vi "UHR-Fleezers Control (host) - 10.4.vi"() -> ()   [LabVIEW 2010] (continued)
            n251 = Absolute Value(x=w2893) -> (abs(x)=w2881:dbl)
            n252 = Compound Arithmetic op=MULTIPLY(w2899, w2898, w2887) -> (w2894:u64)
            n253 = local write "wait to reset values"(w2909) -> ()
            n254 = local write "MCL Scanning"(w2909) -> ()
            n255 = Divide(x=w2894, y=w2881) -> (x/y=w2891:dbl)
            "MCL Count" <- w2891
            n256 = xnode "Read/Write Control"("FPGA VI Reference In"=w2908, "error in"=w2907, "Scan steps (MCL)"=w2881, "Number of scans (MCL)"=w2903, "Cycles per step (MCL)"=u64 1, "Scan freq.  increment (MCL)"=w2884, "1D or 2D Scan?"=w2904, "MCL Scan Axis"=w2904, "Cont. Scan (MCL)"=w2904, "MCL count"=w2891) -> ("FPGA VI Reference Out"=w2906:T20, "error out"=w2905:errorcluster)
            n257 = xnode "Read/Write Control"("FPGA VI Reference In"=w2906, "error in"=w2905, "AI to FIFO"=w2909, "APD to FIFO"=w2909, "Start scan"=w2909, "Start scan (MCL)"=w2909) -> ("FPGA VI Reference Out"=w2911:T20, "error out"=w2910:errorcluster)
          }
        }
        "Raster Scanning..." <- TRUE ("Scanning...")
      }
    }
    n258 = Subtract(x=w848, y=w853) -> (x-y=→"x-y 2":u32)
    n259 = And(x="Save scans", y=w1057) -> (x .and. y?=w1103:bool)
    n260 = Compound Arithmetic op=OR("Start MCL Scan", "Confocal Image", "Confocal Linescan") -> (w1055:bool)
    n261 = And(x="Save Data (MCL)", y=w1055) -> (x .and. y?=w1102:bool)
    n262 = case "Start MCL raster scan" shown="False" w1055 {
      tunnel: w1105 -> [w2126 w2141]
      tunnel: w1104 -> [w2125 w2140]
      tunnel: [w2126 w2136] -> w861
      tunnel: [w2125 w2135] -> w860
      tunnel: [FALSE w2134] -> w1088
      tunnel: "Start MCL Scan" -> [_ w2129]
      tunnel: "Confocal Image" -> [_ w2128]
      tunnel: "Confocal Linescan" -> [_ _]
      frame False {
      }
      frame True {
        w2134 = TRUE
        n263 = case shown="True" "Restart DMA? (MCL)" {
          tunnel: [w2386 w2388] -> w2139
          tunnel: [w2385 w2387] -> w2138
          tunnel: w2141 -> [w2386 w2391]
          tunnel: w2140 -> [w2385 w2390]
          frame False {
          }
          frame True {
            n264 = call "reset FPGA DMA.vi"("error in"=w2390, "FPGA VI Reference In"=w2391) -> ("error out"=w2387:errorcluster, "FPGA VI Reference Out"=w2388:T20)
            n265 = local write "Overflow (data lost)"(FALSE ("Overflow (data lost)")) -> ()
          }
        }
        n266 = case shown="False" w2129 {
          selector: w2129 -> [_ w2145]
          tunnel: w2128 -> [w2144 _]
          tunnel: [w2144 w2145] -> w2127
          frame False {
            n267 = property on="2D or 1D Scan" class="Bool (strict)"("Val(Sgnl)"=w2144) -> ()  [unwired: 2 in, 2 out]
            n268 = property on="Confocal Image" class="Bool (strict)"("Value"=FALSE ("Start Confocal Map")) -> ()  [unwired: 2 in, 2 out]
          }
          frame True {
          }
        }
        n269 = local write "MCL Scanning"(w2134) -> ()
        n270 = local read "AO1"() -> (w2131:dbl)
        n271 = local read "AO2"() -> (w2130:dbl)
        n272 = case shown="False" "Center Scan" {
          tunnel: w2139 -> [w2152 w2264]
          tunnel: w2138 -> [w2151 w2263]
          tunnel: [w2150 w2262] -> w2136
          tunnel: [w2149 w2261] -> w2135
          tunnel: [w2147 w2248] -> w2133
          tunnel: [w2146 w2247] -> w2132
          tunnel: w2131 -> [w2147 w2253]
          tunnel: w2130 -> [w2146 w2256]
          tunnel: w2127 -> [_ _]
          frame False {
            w2148 = TRUE ("AI to FIFO")
            n273 = xnode "Read/Write Control"("FPGA VI Reference In"=w2152, "error in"=w2151, "AI to FIFO"=w2148, "APD to FIFO"=w2148, "Start scan (MCL)"=w2148) -> ("FPGA VI Reference Out"=w2150:T20, "error out"=w2149:errorcluster)
          }
          frame True {
            w2260 = TRUE ("AI to FIFO")
            n274 = local read "Scan steps (MCL)"() -> (w2239:u64)
            n275 = local read "Scan lines (y)"() -> (w2235:u64)
            n276 = local read "Fast Scan Dir"() -> (w2246:bool)
            n277 = local read "Actual MCL Inc (V)"() -> (w2236:dbl)
            n278 = Decrement(x=w2235) -> (x-1=w2234:u64)
            n279 = Decrement(x=w2239) -> (x-1=w2238:u64)
            n280 = Multiply(x=w2236, y=w2234) -> (x*y=w2233:dbl)
            n281 = Divide(x=w2233, y=2.0) -> (x/y=w2243:dbl)
            n282 = Multiply(x=w2236, y=w2238) -> (x*y=w2237:dbl)
            n283 = Divide(x=w2237, y=2.0) -> (x/y=w2242:dbl)
            n284 = Select(t=w2242, s=w2246, f=w2243) -> (s? t:f=w2241:dbl)
            n285 = Select(t=w2243, s=w2246, f=w2242) -> (s? t:f=w2245:dbl)
            n286 = Subtract(x=w2253, y=w2245) -> (x-y=w2244:dbl)
            n287 = Subtract(x=w2256, y=w2241) -> (x-y=w2240:dbl)
            n288 = local read "2D or 1D Scan"() -> (w2258:bool)
            n289 = Not(x=w2246) -> (.not. x?=w2252:bool)
            n290 = Not(x=w2258) -> (.not. x?=w2254:bool)
            n291 = And(x=w2246, y=w2254) -> (x .and. y?=w2255:bool)
            n292 = And(x=w2254, y=w2252) -> (x .and. y?=w2257:bool)
            n293 = Select(t=w2256, s=w2257, f=w2240) -> (s? t:f=w2247:dbl)
            n294 = Select(t=w2253, s=w2255, f=w2244) -> (s? t:f=w2248:dbl)
            n295 = call "Volt to I16.vi"("Voltage In"=w2248) -> ("I16 Voltage Out"=w2251:i16)
            n296 = call "Volt to I16.vi"("Voltage In"=w2247) -> ("I16 Voltage Out"=w2250:i16)
            n297 = xnode "Read/Write Control"("FPGA VI Reference In"=w2264, "error in"=w2263, "AI to FIFO"=w2260, "APD to FIFO"=w2260, "Start scan (MCL)"=w2260, "AO1"=w2251, "AO2"=w2250) -> ("FPGA VI Reference Out"=w2262:T20, "error out"=w2261:errorcluster)
          }
        }
        "Initial Y" <- w2133
        "Initial X" <- w2132
        "wait to reset values" <- w2134
      }
    }
    n298 = local read "Trap Pos Elements/DMA read"() -> (w936:u32)
    n299 = local read "Trap AI Elements/DMA read"() -> (w859:u32)
    n300 = local read "APD Elements/DMA read"() -> (w979:u32)
    n301 = local read "Trap AI FIFO Depth"() -> (w1152:u32)
    n302 = xnode "Get APD Data"("FPGA VI Reference In"=w861, "error in"=w860, "Number of Elements"=w979, "Timeout (ms)"=-1) -> ("Data"=w978:u32[], "Elements Remaining"=→"APD FIFO Elements Remaining":u32)  [unwired: 2 out]
    n303 = xnode "Invoke Method"("FPGA VI Reference In"=w861, "error in"=w860, "Number of Elements"=w936, "Timeout (ms)"=-1) -> ("Data"=w900:u16[], "Elements Remaining"=→"Trap Pos FIFO El Remaining":u32)  [unwired: 2 out]
    n304 = xnode "Invoke Method"("FPGA VI Reference In"=w861, "error in"=w860, "Number of Elements"=w859, "Timeout (ms)"=-1 ("Timeout")) -> ("FPGA VI Reference Out"=w863:T20, "error out"=w862:errorcluster, "Data"=w865:i16[], "Elements Remaining"=w864:u32)
    "Trap AI FIFO El. Rem." <- w864
    n305 = Subtract(x=w1152, y=u32 0) -> (x-y=w1151:u32)
    n306 = Decimate 1D Array(w900) -> (w897:u16[], w899:u16[], w898:u16[])
    n307 = Divide(x=w864, y=w1151) -> (x/y=w1150:dbl)
    "Buffer Status" <- w1150
    n308 = To Unsigned Long Integer(number=w897) -> (unsigned 32bit integer=w896:u32[])
    n309 = Join Numbers(hi=w899, lo=w898) -> ((hi.lo)=w895:u32[])
    n310 = Equal?(x=w1150, y=1.0) -> (x = y?=w1148:bool)
    n311 = Join Numbers(hi=w896, lo=w895) -> ((hi.lo)=w889:u64[])
    n312 = call "IR AOM word to freq - vec.vi"("Frequency Word In (double vec)"=w889) -> ("Frequency Out"=w935:dbl[])
    n313 = case "Alert buffer overflow" shown="True" w1148 {
      frame False {
      }
      frame True {
        n314 = call <vilib>:"Beep.vi"() -> ()  [unwired: 3 in, 9 out]
        "Overflow (data lost)" <- TRUE ("Overflow (data lost)")
      }
    }
    n315 = Decimate 1D Array(w935) -> (w934:dbl[], w933:dbl[])
    n316 = Build Array(w934, w933) -> (w932:dbl[][])
    n317 = local read "Trap Sets"() -> (w1016:u32)
    n318 = case "Deinterlace trap data, average down PSD" shown="1, Default" w1016 {
      tunnel: w865 -> [w2421 w2486]
      tunnel: [w2418 w2483] -> w1009
      tunnel: [w2421 w2485] -> w892
      tunnel: "Detector Type" -> [w2420 w2481]
      tunnel: [w2419 w2484] -> w1008
      tunnel: [w2417 w2482] -> w1123
      frame 1, Default {
        n319 = Divide(x=w2421, y=3276.7) -> (x/y=w2422:dbl[])
        n320 = Decimate 1D Array(w2422) -> (w2431:dbl[], w2430:dbl[], w2429:dbl[], w2428:dbl[], w2427:dbl[], w2426:dbl[], w2425:dbl[], w2424:dbl[])
        n321 = case shown="\"IR-QPD + PSD + FB-QPD position\"" w2420 {
          tunnel: w2431 -> [w2455 w2480]
          tunnel: w2430 -> [w2454 w2479]
          tunnel: w2429 -> [w2439 w2457]
          tunnel: w2428 -> [w2440 w2467]
          tunnel: w2427 -> [w2453 w2478]
          tunnel: w2426 -> [w2452 w2477]
          tunnel: w2425 -> [w2436 w2458]
          tunnel: w2424 -> [w2435 w2456]
          tunnel: [w2434 w2464] -> w2419
          tunnel: [w2433 w2463] -> w2418
          tunnel: [w2432 w2462] -> w2417
          frame "IR-QPD + PSD + FB-QPD", Default {
            w2432 = 0  # Channel pattern
            n322 = Divide(x=w2455, y=w2440) -> (x/y=w2442:dbl[])
            n323 = Divide(x=w2454, y=w2440) -> (x/y=w2441:dbl[])
            n324 = Divide(x=w2453, y=w2436) -> (x/y=w2438:dbl[])
            n325 = Divide(x=w2452, y=w2435) -> (x/y=w2437:dbl[])
            n326 = Build Array(w2442, w2441, w2440, w2439, w2438, w2437, w2436, w2435) -> (w2433:dbl[][])
            n327 = Bundle("T1 Y", "T1 X", "T1 Sum", "FB Sum", "PSD Y", "PSD X", "PSD Y Sum", "PSD X Sum") -> (w2451:T39)  [unwired: 1 out]
            n328 = Cluster To Array(cluster=w2451) -> (array=w2434:string[])
          }
          frame "IR-QPD + PSD + FB-QPD position" {
            w2462 = 3  # Channel pattern
            n329 = Negate(x=w2458) -> (-x=w2459:dbl[])
            n330 = Divide(x=w2480, y=w2467) -> (x/y=w2469:dbl[])
            n331 = Divide(x=w2479, y=w2467) -> (x/y=w2468:dbl[])
            n332 = Divide(x=w2478, y=w2458) -> (x/y=w2466:dbl[])
            n333 = Divide(x=w2477, y=w2459) -> (x/y=w2465:dbl[])
            n334 = Build Array(w2469, w2468, w2467, w2456, w2457, w2466, w2465, w2458) -> (w2463:dbl[][])
            n335 = Bundle("T1 Y", "T1 X", "T1 Sum", "FB X", "FB Sum", "PSD Y", "PSD X", "PSD Y Sum") -> (w2476:T39)  [unwired: 1 out]
            n336 = Cluster To Array(cluster=w2476) -> (array=w2464:string[])
          }
        }
      }
      frame 2 {
        n337 = case shown="\"IR-QPD + PSD + FB-QPD X position\"" w2481 {
          tunnel: w2486 -> [w2548 w2615 w2686]
          tunnel: [w2487 w2606 w2617] -> w2485
          tunnel: [w2514 w2597 w2664] -> w2484
          tunnel: [w2513 w2560 w2631] -> w2483
          tunnel: [w2507 w2595 w2662] -> w2482
          frame "IR-QPD + PSD + FB-QPD", Default {
            w2507 = 1  # Channel pattern
            # "time average x2 the 4th signal and the 4 psd signals (detection laser)"
            # "deinterlace 3 signals from qpd"
            n338 = Decimate 1D Array(w2548) -> (w2547:i16[], w2546:i16[], w2512:i16[], w2545:i16[], w2535:i16[], w2533:i16[], w2532:i16[], w2530:i16[])
            n339 = Decimate 1D Array(w2512) -> (w2511:i16[], w2510:i16[])
            n340 = Decimate 1D Array(w2547) -> (w2544:i16[], w2516:i16[])
            n341 = Decimate 1D Array(w2546) -> (w2543:i16[], w2541:i16[])
            n342 = Decimate 1D Array(w2545) -> (w2542:i16[], w2540:i16[])
            n343 = call "downsample 1D array - double.vi"("Ave N"=2.0, "Array In"=w2535) -> ("Array Out"=w2534:dbl[])  [unwired: 1 out]
            n344 = call "downsample 1D array - double.vi"("Ave N"=2.0, "Array In"=w2533) -> ("Array Out"=w2515:dbl[])  [unwired: 1 out]
            n345 = call "downsample 1D array - double.vi"("Ave N"=2.0, "Array In"=w2532) -> ("Array Out"=w2531:dbl[])  [unwired: 1 out]
            n346 = call "downsample 1D array - double.vi"("Ave N"=2.0, "Array In"=w2530) -> ("Array Out"=w2529:dbl[])  [unwired: 1 out]
            n347 = Interleave 1D Arrays(w2544, w2543, w2542, w2516, w2541, w2540, w2511, w2510, w2534, w2515, w2531, w2529) -> (w2528:dbl[])
            n348 = Divide(x=w2528, y=3276.7) -> (x/y=w2527:dbl[])
            n349 = Decimate 1D Array(w2527) -> (w2526:dbl[], w2525:dbl[], w2524:dbl[], w2523:dbl[], w2522:dbl[], w2521:dbl[], w2509:dbl[], w2508:dbl[], w2520:dbl[], w2519:dbl[], w2518:dbl[], w2517:dbl[])
            n350 = Divide(x=w2526, y=w2524) -> (x/y=w2494:dbl[])
            n351 = Divide(x=w2525, y=w2524) -> (x/y=w2493:dbl[])
            n352 = Divide(x=w2523, y=w2521) -> (x/y=w2492:dbl[])
            n353 = Divide(x=w2522, y=w2521) -> (x/y=w2491:dbl[])
            n354 = Divide(x=w2520, y=w2518) -> (x/y=w2490:dbl[])
            n355 = Divide(x=w2519, y=w2517) -> (x/y=w2489:dbl[])
            n356 = Build Array(w2494, w2493, w2524, w2492, w2491, w2521, w2509, w2508, w2490, w2489, w2518, w2517) -> (w2513:dbl[][])
            n357 = Bundle("T1 Y", "T1 X", "T1 Sum", "T2 Y", "T2 X", "T2 Sum", "T1 FB Sum", "T2 FB Sum", "PSD Y", "PSD X", "PSD Y Sum", "PSD X Sum") -> (w2495:T40)  [unwired: 1 out]
            n358 = To Word Integer(number=w2528) -> (16bit integer=w2487:i16[])
            n359 = Cluster To Array(cluster=w2495) -> (array=w2514:string[])
          }
          frame "IR-QPD + PSD + FB-QPD X position" {
            w2595 = 2  # Channel pattern
            # "time average x2 the 3 psd signals (detection laser)"
            # "deinterlace 3 signals from qpds"
            n360 = Decimate 1D Array(w2615) -> (w2614:i16[], w2613:i16[], w2596:i16[], w2612:i16[], w2558:i16[], w2555:i16[], w2552:i16[], w2583:i16[])
            n361 = Decimate 1D Array(w2596) -> (w2581:i16[], w2579:i16[])
            n362 = Decimate 1D Array(w2614) -> (w2611:i16[], w2598:i16[])
            n363 = Decimate 1D Array(w2613) -> (w2610:i16[], w2608:i16[])
            n364 = Decimate 1D Array(w2612) -> (w2609:i16[], w2607:i16[])
            n365 = Decimate 1D Array(w2583) -> (w2582:i16[], w2580:i16[])
            n366 = call "downsample 1D array - I16.vi"("Ave N"=2.0, "Array In"=w2558) -> ("Array Out"=w2556:i16[])  [unwired: 1 in]
            n367 = call "downsample 1D array - I16.vi"("Ave N"=2.0, "Array In"=w2552) -> ("Array Out"=w2550:i16[])  [unwired: 1 in]
            n368 = call "downsample 1D array - I16.vi"("Ave N"=2.0, "Array In"=w2555) -> ("Array Out"=w2553:i16[])  [unwired: 1 in]
            n369 = Interleave 1D Arrays(w2611, w2610, w2609, w2598, w2608, w2607, w2582, w2581, w2580, w2579, w2556, w2553, w2550) -> (w2606:i16[])
            n370 = Divide(x=w2606, y=3276.7) -> (x/y=w2605:dbl[])
            n371 = Decimate 1D Array(w2605) -> (w2604:dbl[], w2603:dbl[], w2602:dbl[], w2601:dbl[], w2600:dbl[], w2599:dbl[], w2571:dbl[], w2569:dbl[], w2568:dbl[], w2566:dbl[], w2565:dbl[], w2564:dbl[], w2561:dbl[])
            n372 = Negate(x=w2561) -> (-x=w2559:dbl[])
            n373 = Divide(x=w2565, y=w2561) -> (x/y=w2563:dbl[])
            n374 = Divide(x=w2564, y=w2559) -> (x/y=w2562:dbl[])
            n375 = Divide(x=w2604, y=w2602) -> (x/y=w2587:dbl[])
            n376 = Divide(x=w2603, y=w2602) -> (x/y=w2586:dbl[])
            n377 = Divide(x=w2601, y=w2599) -> (x/y=w2585:dbl[])
            n378 = Divide(x=w2600, y=w2599) -> (x/y=w2584:dbl[])
            n379 = Divide(x=w2571, y=w2569) -> (x/y=w2570:dbl[])
            n380 = Divide(x=w2568, y=w2566) -> (x/y=w2567:dbl[])
            n381 = Build Array(w2587, w2586, w2602, w2585, w2584, w2599, w2570, w2569, w2567, w2566, w2563, w2562, w2561) -> (w2560:dbl[][])
            n382 = Bundle("T1 Y", "T1 X", "T1 Sum", "T2 Y", "T2 X", "T2 Sum", "T1 FB X", "T1 FB Sum", "T2 FB X", "T2 FB Sum", "PSD Y", "PSD X", "PSD Y Sum") -> (w2588:T41)  [unwired: 1 out]
            n383 = Cluster To Array(cluster=w2588) -> (array=w2597:string[])
          }
          frame "IR-QPD + PSD + FB-QPD XY positions" {
            w2662 = 4  # Channel pattern
            # "time average x2 the 3 psd signals (detection laser)"
            # "deinterlace 3 signals from qpds"
            n384 = Decimate 1D Array(w2686) -> (w2685:i16[], w2684:i16[], w2663:i16[], w2683:i16[], w2629:i16[], w2675:i16[], w2674:i16[], w2651:i16[])
            n385 = Decimate 1D Array "Feedback Sum"(w2663) -> (w2647:i16[], w2645:i16[])
            n386 = Decimate 1D Array "QPD Y"(w2685) -> (w2682:i16[], w2665:i16[])
            n387 = Decimate 1D Array "QPD X"(w2684) -> (w2681:i16[], w2679:i16[])
            n388 = Decimate 1D Array "Feedback Y"(w2629) -> (w2628:i16[], w2627:i16[])
            n389 = Decimate 1D Array "QPD Sum"(w2683) -> (w2680:i16[], w2678:i16[])
            n390 = Decimate 1D Array "Feedback X"(w2651) -> (w2648:i16[], w2646:i16[])
            n391 = call "downsample 1D array - double.vi"("Ave N"=2.0, "Array In"=w2675) -> ("Array Out"=w2650:dbl[])  [unwired: 1 out]
            n392 = call "downsample 1D array - double.vi"("Ave N"=2.0, "Array In"=w2674) -> ("Array Out"=w2649:dbl[])  [unwired: 1 out]
            n393 = Interleave 1D Arrays(w2682, w2681, w2680, w2665, w2679, w2678, w2628, w2648, w2647, w2627, w2646, w2645, w2650, w2649) -> (w2673:dbl[])
            n394 = Divide(x=w2673, y=3276.7) -> (x/y=w2672:dbl[])
            n395 = Decimate 1D Array(w2672) -> (w2671:dbl[], w2670:dbl[], w2669:dbl[], w2668:dbl[], w2667:dbl[], w2666:dbl[], w2624:dbl[], w2638:dbl[], w2622:dbl[], w2623:dbl[], w2636:dbl[], w2620:dbl[], w2634:dbl[], w2632:dbl[])
            n396 = Negate(x=w2632) -> (-x=w2630:dbl[])
            n397 = Divide(x=w2634, y=w2630) -> (x/y=w2633:dbl[])
            n398 = Divide(x=w2623, y=w2620) -> (x/y=w2619:dbl[])
            n399 = Divide(x=w2624, y=w2622) -> (x/y=w2621:dbl[])
            n400 = Divide(x=w2671, y=w2669) -> (x/y=w2655:dbl[])
            n401 = Divide(x=w2670, y=w2669) -> (x/y=w2654:dbl[])
            n402 = Divide(x=w2668, y=w2666) -> (x/y=w2653:dbl[])
            n403 = Divide(x=w2667, y=w2666) -> (x/y=w2652:dbl[])
            n404 = Divide(x=w2638, y=w2622) -> (x/y=w2637:dbl[])
            n405 = Divide(x=w2636, y=w2620) -> (x/y=w2635:dbl[])
            n406 = Build Array(w2655, w2654, w2669, w2653, w2652, w2666, w2621, w2637, w2622, w2619, w2635, w2620, w2633, w2632) -> (w2631:dbl[][])
            n407 = Bundle("T1 Y", "T1 X", "T1 Sum", "T2 Y", "T2 X", "T2 Sum", "T1 FB Y", "T1 FB X", "T1 FB Sum", "T2 FB Y", "T2 FB X", "T2 FB Sum", "PSD X", "PSD Y Sum") -> (w2618:T42)  [unwired: 1 out]
            n408 = To Word Integer(number=w2673) -> (16bit integer=w2617:i16[])
            n409 = Cluster To Array(cluster=w2618) -> (array=w2664:string[])
          }
        }
      }
    }
    "AI labels" <- w1008
    n410 = Decimate 1D Array(w978) -> (w1006:u32[], w942:u32[])
    n411 = local read "DMA Update Period (s)"() -> (w1017:dbl)
    n412 = local read "BD 1 Frequency 2 (MHz)"() -> (w884:dbl)
    n413 = local read "BD 1 Frequency 1 (MHz)"() -> (w885:dbl)
    n414 = Build Array(w1006, w942) -> (w1085:u32[][])
    n415 = local read "Data Period (s)"() -> (w991:dbl)
    n416 = Decimate 1D Array(w892) -> (w915:i16[], w914:i16[], w912:i16[], w911:i16[])  [unwired: 9 out]
    n417 = To Double Precision Float(number=w1085) -> (double precision float=w1086:dbl[][])
    n418 = local read "APD Integration Time (s)"() -> (w955:dbl)
    n419 = Divide(x=w915, y=w914) -> (x/y=w916:dbl[])
    n420 = Divide(x=w912, y=w911) -> (x/y=w913:dbl[])
    n421 = feedback #1(0.0) -> (w929:dbl)
    n422 = Add(x=w1017, y=w929) -> (x+y=w1125:dbl)
    n423 = feedback-in #1(w1125) -> ()
    n424 = local read "AOM X Cal (nm/MHz)"() -> (w882:dbl)
    n425 = To Time Stamp(1:w929) -> (0:w928:timestamp)
    n426 = Split 1D Array(array=w916, index="N El. to Ave.") -> (second subarray=w919:dbl[])  [unwired: 1 out]
    n427 = Split 1D Array(array=w913, index="N El. to Ave.") -> (second subarray=w918:dbl[])  [unwired: 1 out]
    n428 = local read "Trap X AI1 (DMA)"() -> (w917:T14)
    n429 = Multiply(x=w991, y="Trap Disp. Downsample") -> (x*y=w930:dbl)
    "Display Period (s)" <- w930
    n430 = Bundle("BD 1 Frequency 1 (MHz)"=w885, "BD 1 Frequency 2 (MHz)"=w884) -> (w886:T43)  [unwired: 1 out]
    n431 = for "Trap AI" {
      tunnel: [w2416] -> w1119 mode=indexing
      tunnel: w928 -> [w2406]
      tunnel: "Trap Disp. Downsample" -> [w2414]
      tunnel: w1009 -> [w2412] mode=indexing
      tunnel: w991 -> [w2411]
      tunnel: w1008 -> [w2410] mode=indexing
      tunnel: w927 -> [w2409]
      tunnel: [w2408] -> w966 mode=indexing
      tunnel: w930 -> [w2407]
      workers-P: _ -> [_]
      n432 = Bundle By Name("Y"=w2412, "dt"=w2411) -> (w2413:waveform(dbl))  [unwired: 1 out]
      n433 = Set Waveform Attribute(5:w2410, 6:w2409, 7:w2413) -> (3:w2408:waveform(dbl))  [unwired: 1 in, 2 out]
      n434 = call "downsample 1D array - double.vi"("Ave N"=w2414, "Array In"=w2412) -> ("Array Out"=w2415:dbl[])  [unwired: 1 out]
      n435 = Bundle By Name(cluster=w2408, "t0"=w2406, "Y"=w2415, "dt"=w2407) -> (w2416:waveform(dbl))
    }
    n436 = call <vilib>:"Mean.vi"("X"=w918) -> ("mean"=w906:dbl)  [unwired: 1 out]
    n437 = call <vilib>:"Mean.vi"("X"=w919) -> ("mean"=w907:dbl)  [unwired: 1 out]
    n438 = Cluster To Array(cluster=w886) -> (array=w883:dbl[])
    n439 = Reciprocal(x=w930) -> (1/x=→"Trap Disp. Freq. (Hz)":dbl)
    n440 = local read "Data points/scans (MCL)"() -> (w1097:dbl)
    n441 = To Fixed-Point(number=w906) -> (fixed-point=w904:fxp<+/-,16,1>)  [unwired: 1 in]
    n442 = To Fixed-Point(number=w907) -> (fixed-point=w905:fxp<+/-,16,1>)  [unwired: 1 in]
    n443 = Bundle("Trap 1 Pos.", "Trap 2 Pos.") -> (w926:cluster{string, string})  [unwired: 1 out]
    n444 = Bundle By Name(cluster=w917, "Set 1"=w905, "Set 2"=w904) -> (→"Trap X AI1 (DMA)":T14)
    n445 = Cluster To Array(cluster=w926) -> (array=w923:string[])
    n446 = for "Trap Position" {
      tunnel: w932 -> [w1321] mode=indexing
      tunnel: "Trap Disp. Downsample" -> [w1320]
      tunnel: w930 -> [w1318]
      tunnel: w928 -> [w1317]
      tunnel: w927 -> [w1315]
      tunnel: w923 -> [w1314] mode=indexing
      tunnel: [w1313] -> w881 mode=indexing
      tunnel: w883 -> [w1311] mode=indexing
      tunnel: w882 -> [w1309]
      n447 = call "downsample 1D array - double.vi"("Ave N"=w1320, "Array In"=w1321) -> ("Array Out"=w1319:dbl[])  [unwired: 1 out]
      n448 = Subtract(x=w1319, y=w1311) -> (x-y=w1312:dbl[])
      n449 = Multiply(x=w1309, y=w1312) -> (x*y=w1310:dbl[])
      n450 = Bundle By Name("Y"=w1310, "dt"=w1318, "t0"=w1317) -> (w1316:waveform(dbl))  [unwired: 1 out]
      n451 = Set Waveform Attribute(5:w1314, 6:w1315, 7:w1316) -> (3:w1313:waveform(dbl))  [unwired: 1 in, 2 out]
    }
    "Trap Positions" <- w881
    n452 = Bundle("APD 1", "APD 2") -> (w1118:cluster{string, string})  [unwired: 1 out]
    n453 = Cluster To Array(cluster=w1118) -> (array=w1115:string[])
    n454 = for "APD" {
      tunnel: w1086 -> [w2395] mode=indexing
      tunnel: w955 -> [w2403]
      tunnel: [w2399] -> w962 mode=indexing
      tunnel: "APD Disp. Scale" -> [w2400]
      tunnel: w927 -> [w2398]
      tunnel: w1115 -> [w2397] mode=indexing
      tunnel: "APD Disp. Downsample" -> [w2393]
      tunnel: [w2396] -> w1114
      workers-P: _ -> [_]
      tunnel: w928 -> [w2392]
      n455 = call "integrate 1D array interval - double.vi"("Ave N"=w2393, "Array In"=w2395) -> ("Array Out"=w2394:dbl[])  [unwired: 1 out]
      n456 = Multiply(x=w2403, y=w2393) -> (x*y=w2396:dbl)
      n457 = Divide(x=w2394, y=w2400) -> (x/y=w2401:dbl[])
      n458 = Bundle By Name("t0"=w2392, "Y"=w2401, "dt"=w2396) -> (w2402:waveform(dbl))  [unwired: 1 out]
      n459 = Set Waveform Attribute(5:w2397, 6:w2398, 7:w2402) -> (3:w2399:waveform(dbl))  [unwired: 1 in, 2 out]
    }
    "APD Display Period (s)" <- w1114
    n460 = Reciprocal(x=w1114) -> (1/x=→"APD Display Freq. (Hz)":dbl)
    n461 = local read "Display Period (s)"() -> (w990:dbl)
    n462 = Increment(x=w1097) -> (x+1=w1098:dbl)
    n463 = Index Array(array=w881, index=0) -> (element=w879:waveform(dbl))
    n464 = To Double Precision Float(number=w1006) -> (double precision float=w1005:dbl[])
    n465 = feedback #2(w1098) -> (w1101:dbl)
    n466 = Select(t=0, s=w1088, f=w1101) -> (s? t:f=w1094:dbl)
    n467 = Array Size(array=w1005) -> (size(s)=w1100:i32)
    n468 = Add(x=w1100, y=w1094) -> (x+y=w1095:dbl)
    n469 = Unbundle By Name(w879) -> ("Y"=w877:dbl[])
    n470 = feedback #3(w1006) -> (w1084:u32[])
    n471 = Build Array (concatenate)(w1084, w1006) -> (w1081:u32[])
    n472 = feedback #4(w942) -> (w961:u32[])
    n473 = Divide(x="Bead Sep. Int. Time (s)", y=w990) -> (x/y=w875:dbl)
    n474 = Build Array (concatenate)(w961, w942) -> (w960:u32[])
    n475 = Greater?(x=w1095, y=w1097) -> (0:w1096:bool)
    n476 = feedback #5(w877) -> (w878:dbl[])
    n477 = Build Array (concatenate)(w877, w878) -> (w876:dbl[])
    n478 = Select(t=w1094, s=w1096, f=w1095) -> (s? t:f=w1093:dbl)
    n479 = feedback-in #2(w1093) -> ()
    n480 = Array Size(array=w1081) -> (size(s)=w1078:i32)
    n481 = Array Size(array=w1006) -> (size(s)=w1080:i32)
    n482 = local read "MCL Scanning"() -> (w1091:bool)
    n483 = local read "APD Integration Time (s)"() -> (w969:dbl)
    n484 = Build Array (concatenate)(w962, w1119) -> (w964:waveform(dbl)[])
    "All Signals" <- w964
    n485 = Split 1D Array(array=w876, index=w875) -> (first subarray=w869:dbl[])  [unwired: 1 out]
    n486 = feedback-in #5(w869) -> ()
    n487 = Multiply(x=w1080, y="APD Ave N") -> (x*y=w1079:dbl)
    n488 = Greater?(x=w1078, y=w1079) -> (0:w1082:bool)
    n489 = Not(x=w1096) -> (.not. x?=w1090:bool)
    n490 = To Double Precision Float(number=w942) -> (double precision float=w941:dbl[])
    n491 = call <vilib>:"Mean.vi"("X"=w869) -> ("mean"=w868:dbl)  [unwired: 1 out]
    "Mean T1 Position (nm)" <- w868
    n492 = Subtract(x=w869, y=w868) -> (x-y=w874:dbl[])
    n493 = Square(x=w874) -> (x^2=w873:dbl[])
    n494 = And(x=w1090, y=w1091) -> (x .and. y?=w1092:bool)
    n495 = call <vilib>:"Mean.vi"("X"=w873) -> ("mean"=w872:dbl)  [unwired: 1 out]
    n496 = case shown="True" w1082 {
      tunnel: w1081 -> [w1976 w1983]
      tunnel: [w1976 w1981] -> w1022
      tunnel: w1079 -> [_ w1978]
      tunnel: w1078 -> [_ w1982]
      tunnel: w960 -> [w1975 w1980]
      tunnel: [w1975 w1977] -> w957
      frame False {
      }
      frame True {
        n497 = Subtract(x=w1982, y=w1978) -> (x-y=w1979:dbl)
        n498 = Array Subset(array=w1983, index=w1979, length=w1978) -> (w1981:u32[])
        n499 = Array Subset(array=w1980, index=w1979, length=w1978) -> (w1977:u32[])
      }
    }
    n500 = feedback-in #3(w1022) -> ()
    n501 = feedback-in #4(w957) -> ()
    n502 = Or(x=w1092, y=w1088) -> (x .or. y?=w1089:bool)
    n503 = Square Root(x=w872) -> (sqrt(x)=w871:dbl)
    n504 = Equal?(x="Tab Control 6", y=T30."High Res Display") -> (x = y?=w1012:bool)
    n505 = Multiply(x="APD Disp. Scale", y=w962) -> (x*y=w971:waveform(dbl)[])
    n506 = Multiply(x="APD Disp. Downsample", y=w969) -> (x*y=w967:dbl)
    n507 = Multiply(x=10.0, y=w871) -> (x*y=→"Trap 1 Position RMS (A)":dbl)
    n508 = Divide(x=w971, y=w967) -> (x/y=w939:waveform(dbl)[])
    n509 = Index Array(array=w939, index=0) -> (element=w949:waveform(dbl))
    n510 = case "For computing FFTs for display" shown="True" "Compute FFT" {
      tunnel: w966 -> [_ w3239]
      frame False {
      }
      frame True {
        n511 = Build Array("FFT 1 Choice 1", "FFT 1 Choice 2", "FFT 2 Choice 1", "FFT 2 Choice 2") -> (w3232:u16[])
        n512 = Array Size(array=w3239) -> (size(s)=w3238:i32)
        n513 = feedback-in #6(w3232) -> ()
        n514 = feedback #6(u16[] [100, 100, 100, 100]) -> (w3233:u16[])
        n515 = feedback-in #7("# Spectra to Ave.") -> ()
        n516 = feedback #7("# Spectra to Ave.") -> (w3230:dbl)
        n517 = Not Equal?(x="# Spectra to Ave.", y=w3230) -> (x != y?=w3229:bool)
        n518 = Not Equal?(x=w3232, y=w3233) -> (x != y?=w3231:bool)
        n519 = feedback #8(1.0) -> (w3216:dbl)
        n520 = Compound Arithmetic op=OR("Reset FFT", w3231, w3229) -> (w3214:bool)
        n521 = Select(t=1.0, s=w3214, f=w3216) -> (s? t:f=w3218:dbl)
        n522 = Greater?(x=w3218, y="# Spectra to Ave.") -> (0:w3237:bool)
        n523 = Increment(x=w3218) -> (x+1=w3217:dbl)
        n524 = feedback-in #8(w3217) -> ()
        n525 = local read "DMA Update Period (s)"() -> (w3212:dbl)
        n526 = Multiply(x="# Spectra to Ave.", y=w3212) -> (x*y=→"Ave. Time (s)":dbl)
        n527 = Build Array(cluster{"f0":dbl, "df":dbl, "magnitude":dbl[]} {"f0"=0.0, "df"=0.0, "magnitude"=[]} ("PSD")) -> (w3221:cluster{"f0":dbl, "df":dbl, "magnitude":dbl[]}[])
        n528 = Build Array(w3221, w3221, w3221, w3221) -> (w3223:T44)
        n529 = feedback #9(w3223) -> (w3228:T44)
        n530 = for {
          N: 4 -> [_]
          tunnel: w3232 -> [w3261] mode=indexing
          tunnel: w3239 -> [w3262]
          tunnel: w3238 -> [w3264]
          tunnel: w3214 -> [w3257]
          tunnel: w3237 -> [w3256]
          tunnel: "# Spectra to Ave." -> [w3255]
          tunnel: [w3254] -> w3227 mode=indexing
          tunnel: w3228 -> [w3259] mode=indexing
          tunnel: [w3258] -> w3215 mode=indexing
          tunnel: w3218 -> [w3253]
          n531 = Less?(x=w3261, y=w3264) -> (x < y?=w3263:bool)
          n532 = Index Array(array=w3262, index=w3261) -> (element=w3260:waveform(dbl))
          n533 = case shown="True" w3263 {
            tunnel: w3260 -> [_ w3281]
            tunnel: w3259 -> [w3266 w3279]
            tunnel: [w3266 w3267] -> w3258
            tunnel: w3257 -> [_ w3278]
            tunnel: w3256 -> [_ w3271]
            tunnel: w3255 -> [_ w3270]
            tunnel: [cluster{"f0":dbl, "df":dbl, "magnitude":dbl[]} {"f0"=0.0, "df"=0.0, "magnitude"=[]} ("PSD") w3272] -> w3254
            tunnel: w3253 -> [_ w3269]
            frame False {
            }
            frame True {
              n534 = call <vilib>:"Std Deviation and Variance.vi"("X"=w3281) -> ("mean"=w3282:dbl)  [unwired: 1 in, 2 out]
              n535 = Subtract(x=w3281, y=w3282) -> (x-y=w3280:waveform(dbl))
              n536 = xnode "Spectral Measurements"("Signals"=w3280) -> ("PSD"=w3274:cluster{"f0":dbl, "df":dbl, "magnitude":dbl[]})  [unwired: 1 in, 1 out]
              n537 = case shown="False" w3278 {
                tunnel: w3279 -> [w3291 _]
                tunnel: [w3287 w3296] -> w3267
                tunnel: w3274 -> [w3290 w3297]
                tunnel: w3271 -> [w3289 _]
                frame False {
                  n538 = Build Array (concatenate)(w3291, w3290) -> (w3288:cluster{"f0":dbl, "df":dbl, "magnitude":dbl[]}[])
                  n539 = case shown="True" w3289 {
                    tunnel: w3288 -> [w3292 w3295]
                    tunnel: [w3292 w3293] -> w3287
                    frame False {
                    }
                    frame True {
                      n540 = Delete From Array(array=w3295, index=0) -> (array with subset deleted=w3293:cluster{"f0":dbl, "df":dbl, "magnitude":dbl[]}[])  [unwired: 1 in, 1 out]
                    }
                  }
                }
                frame True {
                  n541 = Build Array(w3297) -> (w3296:cluster{"f0":dbl, "df":dbl, "magnitude":dbl[]}[])
                }
              }
              n542 = for {
                tunnel: w3267 -> [w3286] mode=indexing
                tunnel: [w3285] -> w3277 mode=indexing
                workers-P: _ -> [_]
                n543 = Unbundle By Name(w3286) -> ("magnitude"=w3285:dbl[])
              }
              n544 = Transpose 2D Array(2D array=w3277) -> (transposed array=w3276:dbl[][])
              n545 = for {
                tunnel: w3276 -> [w3284] mode=indexing
                tunnel: [w3283] -> w3275 mode=indexing
                workers-P: _ -> [_]
                n546 = Add Array Elements(numeric array=w3284) -> (sum=w3283:dbl)
              }
              n547 = Select(t=w3270, s=w3271, f=w3269) -> (s? t:f=w3268:dbl)
              n548 = Divide(x=w3275, y=w3268) -> (x/y=w3273:dbl[])
              n549 = Bundle By Name(cluster=w3274, "magnitude"=w3273) -> (w3272:cluster{"f0":dbl, "df":dbl, "magnitude":dbl[]})
            }
          }
        }
        n550 = case shown="True" w3214 {
          tunnel: w3215 -> [w3246 w3252]
          tunnel: [w3246 w3247] -> w3213
          frame False {
          }
          frame True {
            n551 = Array Subset(array=w3252, index (row)=0 ("index"), length (row)=4 ("length"), index (col)=0 ("index"), length (col)=1 ("length")) -> (w3247:T44)
          }
        }
        n552 = feedback-in #9(w3213) -> ()
        n553 = Split 1D Array(array=w3227, index=2) -> (first subarray=→"FFT 1":cluster{"f0":dbl, "df":dbl, "magnitude":dbl[]}[], second subarray=→"FFT 2":cluster{"f0":dbl, "df":dbl, "magnitude":dbl[]}[])
      }
    }
    n554 = Index Array(array=w939, index=1) -> (element=w947:waveform(dbl))
    n555 = case "For displaying the high resolution display (no downsampling)" shown="True" w1012 {
      tunnel: w966 -> [_ w1485]
      frame False {
      }
      frame True {
        n556 = Index Array(array=w1485, index="High Res. Display") -> (element=w1486:waveform(dbl))
        n557 = call <vilib>:"Std Deviation and Variance.vi"("X"=w1486) -> ("mean"=w1493:dbl, "standard deviation"=w1498:dbl)  [unwired: 1 in, 1 out]
        "Mean Intensity" <- w1493
        "Sigma" <- w1498
        n558 = Subtract(x=w1486, y=w1493) -> (x-y=w1492:waveform(dbl))
        n559 = Select(t=w1492, s="Subtract mean", f=w1486) -> (s? t:f=→"1 Channel":waveform(dbl))
        n560 = Divide(x=w1498, y=w1493) -> (x/y=→"Sigma/Mean":dbl)
        n561 = feedback #10(1) -> (w1487:i32)
        n562 = Greater Or Equal?(x=w1487, y="Slow mean N ave.") -> (x >= y?=w1500:bool)
        n563 = Increment(x=w1487) -> (x+1=w1502:i32)
        n564 = Select(t=1, s=w1500, f=w1502) -> (s? t:f=w1489:i32)
        n565 = feedback-in #10(w1489) -> ()
        n566 = feedback #11() -> (w1490:waveform(dbl))  [unwired: 1 out]
        n567 = case shown="Default" w1487 {
          tunnel: [w1505 w1508] -> w1491
          tunnel: w1490 -> [w1507 _]
          tunnel: w1486 -> [w1506 w1508]
          frame Default {
            n568 = call-poly <vilib>:"Append Waveforms.vi"("waveform B"=w1506, "waveform A"=w1507) -> ("waveform out"=w1505:waveform(dbl))  [unwired: 1 in, 8 out]
          }
          frame 1 {
          }
        }
        n569 = feedback-in #11(w1491) -> ()
        n570 = case shown="True" w1500 {
          tunnel: w1491 -> [_ w1504]
          frame False {
          }
          frame True {
            n571 = call <vilib>:"Mean.vi"("X"=w1504) -> ("mean"=→"Slow mean":dbl)  [unwired: 1 out]
          }
        }
      }
    }
    n572 = case "For plotting results of scanning MCL" shown="True" w1089 {
      tunnel: w1088 -> [_ w2016]
      tunnel: w1005 -> [_ w2112]
      tunnel: w1097 -> [_ _]
      tunnel: w966 -> [_ w2086]
      tunnel: w941 -> [_ w2017]
      tunnel: w940 -> [_ w1990]
      frame False {
      }
      frame True {
        w1997 = u32 0 items=["Horizontal", "Vertical", "Central", "1st Diagonal", "2nd Diagonal"] ("Type of Symmetry")
        w2025 = u32 0 items=["Horizontal", "Vertical", "Central", "1st Diagonal", "2nd Diagonal"] ("Type of Symmetry")
        w2028 = u32 0 items=["Horizontal", "Vertical", "Central", "1st Diagonal", "2nd Diagonal"] ("Type of Symmetry")
        w2057 = u32 0 items=["Horizontal", "Vertical", "Central", "1st Diagonal", "2nd Diagonal"] ("Type of Symmetry")
        n573 = Index Array(array=w2086, index=10) -> (element=w2092:waveform(dbl))
        n574 = Index Array(array=w2086, index=11) -> (element=w2089:waveform(dbl))
        n575 = local read "Cycles/step (MCL)"() -> (w2042:u64)
        n576 = Index Array(array=w2086, index="Channel") -> (element=w2088:waveform(dbl))
        n577 = Unbundle(w1990) -> ("New Image"=w1989:T2, "New Image"=w1988:T2, "New Image"=w1987:T2, "New Image"=w1986:T2)
        n578 = Unbundle By Name(w2092) -> ("Y"=w2044:dbl[])
        n579 = Unbundle By Name(w2089) -> ("Y"=w2046:dbl[])
        n580 = Unbundle By Name(w2088) -> ("Y"=w2051:dbl[])
        n581 = call "downsample 1D array - double.vi"("Ave N"=w2042, "Array In"=w2044) -> ("Array Out"=w2043:dbl[])  [unwired: 1 out]
        n582 = call "downsample 1D array - double.vi"("Ave N"=w2042, "Array In"=w2046) -> ("Array Out"=w2045:dbl[])  [unwired: 1 out]
        n583 = call "downsample 1D array - double.vi"("Ave N"=w2042, "Array In"=w2051) -> ("Array Out"=w2050:dbl[])  [unwired: 1 out]
        n584 = feedback #12(w2112) -> (w2113:dbl[])
        n585 = Build Array (concatenate)(w2113, w2112) -> (w2094:dbl[])
        n586 = feedback #13(w2017) -> (w2019:dbl[])
        n587 = Build Array (concatenate)(w2019, w2017) -> (w2018:dbl[])
        n588 = local read "Scan steps (MCL)"() -> (w1999:u64)
        n589 = Select(t=w2112, s=w2016, f=w2094) -> (s? t:f=w2098:dbl[])
        n590 = feedback-in #12(w2098) -> ()
        n591 = Select(t=w2017, s=w2016, f=w2018) -> (s? t:f=w2000:dbl[])
        n592 = feedback-in #13(w2000) -> ()
        n593 = local read "Scan lines (y)"() -> (w1985:u64)
        n594 = local read "N APD Samp/step"() -> (w2001:dbl)
        n595 = feedback #14(w2043) -> (w2100:dbl[])
        n596 = Build Array (concatenate)(w2100, w2043) -> (w2091:dbl[])
        n597 = feedback #15(w2050) -> (w2110:dbl[])
        n598 = Build Array (concatenate)(w2110, w2050) -> (w2109:dbl[])
        n599 = feedback #16(w2045) -> (w2102:dbl[])
        n600 = Build Array (concatenate)(w2102, w2045) -> (w2103:dbl[])
        n601 = Select(t=w2043, s=w2016, f=w2091) -> (s? t:f=w2047:dbl[])
        n602 = feedback-in #14(w2047) -> ()
        n603 = Select(t=w2050, s=w2016, f=w2109) -> (s? t:f=w2049:dbl[])
        n604 = feedback-in #15(w2049) -> ()
        n605 = Select(t=w2045, s=w2016, f=w2103) -> (s? t:f=w2048:dbl[])
        n606 = feedback-in #16(w2048) -> ()
        n607 = Multiply(x=w1999, y=u64 2) -> (x*y=w1984:u64)
        n608 = call "integrate 1D array interval - double.vi"("Ave N"=w2001, "Array In"=w2000) -> ("Array Out"=w2012:dbl[])  [unwired: 1 out]
        n609 = call "integrate 1D array interval - double.vi"("Ave N"=w2001, "Array In"=w2098) -> ("Array Out"=w2097:dbl[])  [unwired: 1 out]
        n610 = Array Size(array=w2012) -> (size(s)=w2013:i32)
        n611 = Array Size(array=w2097) -> (size(s)=w2099:i32)
        n612 = Multiply(x=w1985, y=w1984) -> (x*y=w2015:u64)
        n613 = Multiply(x=w1985, y=w1984) -> (x*y=w2107:u64)
        n614 = call <vilib>:"Mean.vi"("X"=w2047) -> ("mean"=w2031:dbl)  [unwired: 1 out]
        n615 = Subtract(x=w2015, y=w2013) -> (x-y=w2006:u64)
        n616 = call <vilib>:"Mean.vi"("X"=w2049) -> ("mean"=w2036:dbl)  [unwired: 1 out]
        n617 = call <vilib>:"Mean.vi"("X"=w2048) -> ("mean"=w2034:dbl)  [unwired: 1 out]
        n618 = call <vilib>:"Mean.vi"("X"=w2012) -> ("mean"=w2003:dbl)  [unwired: 1 out]
        n619 = Subtract(x=w2107, y=w2099) -> (x-y=w2041:u64)
        n620 = call <vilib>:"Mean.vi"("X"=w2097) -> ("mean"=w2038:dbl)  [unwired: 1 out]
        n621 = Initialize Array(1.0 ("element"), w2006) -> (w2002:dbl[])
        n622 = Initialize Array(1.0 ("element"), w2041) -> (w2032:dbl[])
        n623 = Multiply(x=w2002, y=w2003) -> (x*y=w2004:dbl[])
        n624 = Multiply(x=w2032, y=w2034) -> (x*y=w2035:dbl[])
        n625 = Multiply(x=w2032, y=w2036) -> (x*y=w2037:dbl[])
        n626 = Multiply(x=w2032, y=w2031) -> (x*y=w2033:dbl[])
        n627 = Multiply(x=w2032, y=w2038) -> (x*y=w2039:dbl[])
        n628 = Build Array (concatenate)(w2047, w2033) -> (w2101:dbl[])
        n629 = Build Array (concatenate)(w2049, w2037) -> (w2105:dbl[])
        n630 = Build Array (concatenate)(w2048, w2035) -> (w2104:dbl[])
        n631 = Build Array (concatenate)(w2012, w2004) -> (w2014:dbl[])
        n632 = Build Array (concatenate)(w2097, w2039) -> (w2106:dbl[])
        n633 = Reshape Array(w2101, w1985, w1984) -> (w2067:dbl[][])
        n634 = Reshape Array(w2014, w1985, w1984) -> (w2010:dbl[][])
        n635 = Reshape Array(w2105, w1985, w1984) -> (w2059:dbl[][])
        n636 = Reshape Array(w2104, w1985, w1984) -> (w2074:dbl[][])
        n637 = Reshape Array(w2106, w1985, w1984) -> (w2084:dbl[][])
        n638 = Array Subset(array=w2074, index (col)=0 ("index"), length (col)=w1999) -> (w2079:dbl[][])  [unwired: 2 in]
        n639 = Array Subset(array=w2074, index (col)=w1999) -> (w2077:dbl[][])  [unwired: 3 in]
        n640 = Array Subset(array=w2059, index (col)=0 ("index"), length (col)=w1999) -> (w2065:dbl[][])  [unwired: 2 in]
        n641 = Array Subset(array=w2059, index (col)=w1999) -> (w2063:dbl[][])  [unwired: 3 in]
        n642 = Array Subset(array=w2010, index (col)=0 ("index"), length (col)=w1999) -> (w2009:dbl[][])  [unwired: 2 in]
        n643 = Array Subset(array=w2010, index (col)=w1999) -> (w2007:dbl[][])  [unwired: 3 in]
        n644 = Array Subset(array=w2084, index (col)=0 ("index"), length (col)=w1999) -> (w2083:dbl[][])  [unwired: 2 in]
        n645 = Array Subset(array=w2084, index (col)=w1999) -> (w2081:dbl[][])  [unwired: 3 in]
        n646 = Array Subset(array=w2067, index (col)=0 ("index"), length (col)=w1999) -> (w2072:dbl[][])  [unwired: 2 in]
        n647 = Array Subset(array=w2067, index (col)=w1999) -> (w2070:dbl[][])  [unwired: 3 in]
        n648 = for {
          tunnel: w2079 -> [w2121] mode=indexing
          tunnel: [w2120] -> w2078 mode=indexing
          workers-P: _ -> [_]
          n649 = Reverse 1D Array(array=w2121) -> (reversed array=w2120:dbl[])
        }
        n650 = for {
          tunnel: w2065 -> [w2117] mode=indexing
          tunnel: [w2116] -> w2064 mode=indexing
          workers-P: _ -> [_]
          n651 = Reverse 1D Array(array=w2117) -> (reversed array=w2116:dbl[])
        }
        n652 = for {
          tunnel: w2009 -> [w2115] mode=indexing
          tunnel: [w2114] -> w2008 mode=indexing
          workers-P: _ -> [_]
          n653 = Reverse 1D Array(array=w2115) -> (reversed array=w2114:dbl[])
        }
        n654 = for {
          tunnel: w2083 -> [w2123] mode=indexing
          tunnel: [w2122] -> w2082 mode=indexing
          workers-P: _ -> [_]
          n655 = Reverse 1D Array(array=w2123) -> (reversed array=w2122:dbl[])
        }
        n656 = for {
          tunnel: w2072 -> [w2119] mode=indexing
          tunnel: [w2118] -> w2071 mode=indexing
          workers-P: _ -> [_]
          n657 = Reverse 1D Array(array=w2119) -> (reversed array=w2118:dbl[])
        }
        n658 = Index Array(array=w2084, index (row)=0) -> (element=→"Waveform Graph":dbl[])  [unwired: 1 in]
        n659 = Add(x=w2078, y=w2077) -> (x+y=w2076:dbl[][])
        n660 = Add(x=w2064, y=w2063) -> (x+y=w2062:dbl[][])
        n661 = Add(x=w2008, y=w2007) -> (x+y=w1992:dbl[][])
        n662 = Add(x=w2082, y=w2081) -> (x+y=w2056:dbl[][])
        n663 = Add(x=w2071, y=w2070) -> (x+y=w2069:dbl[][])
        n664 = Divide(x=w2062, y=2) -> (x/y=w2060:dbl[][])
        n665 = Divide(x=w2076, y=2) -> (x/y=w2021:dbl[][])
        n666 = Divide(x=w2069, y=2) -> (x/y=w2023:dbl[][])
        n667 = To Single Precision Float(number=w2056) -> (single precision float=w2055:sgl[][])
        n668 = Transpose 2D Array(2D array=w2060) -> (transposed array=→"Data map":dbl[][])
        n669 = To Single Precision Float(number=w1992) -> (single precision float=w1996:sgl[][])
        n670 = To Single Precision Float(number=w2021) -> (single precision float=w2027:sgl[][])
        n671 = To Single Precision Float(number=w2023) -> (single precision float=w2024:sgl[][])
        n672 = call "IMAQ ArrayToImage"("Image Pixels (Float)"=w2055, "Image"=w1989) -> ("Image Out"=w2058:T2)  [unwired: 8 in, 1 out]
        n673 = call "IMAQ ArrayToImage"("Image Pixels (Float)"=w1996, "Image"=w1988) -> ("Image Out"=w1998:T2)  [unwired: 8 in, 1 out]
        n674 = call "IMAQ ArrayToImage"("Image Pixels (Float)"=w2027, "Image"=w1987) -> ("Image Out"=w2029:T2)  [unwired: 8 in, 1 out]
        n675 = call "IMAQ ArrayToImage"("Image Pixels (Float)"=w2024, "Image"=w1986) -> ("Image Out"=w2026:T2)  [unwired: 8 in, 1 out]
        n676 = call "IMAQ Symmetry"("Type of Symmetry"=w2057, "Image Src"=w2058) -> ("Image Dst Out"=w2053:T2)  [unwired: 3 in, 1 out]
        n677 = call "IMAQ Symmetry"("Type of Symmetry"=w1997, "Image Src"=w1998) -> ("Image Dst Out"=w1994:T2)  [unwired: 3 in, 1 out]
        n678 = call "IMAQ Symmetry"("Type of Symmetry"=w2028, "Image Src"=w2029) -> ("Image Dst Out"=→"Detection Laser X":T2)  [unwired: 3 in, 1 out]
        n679 = call "IMAQ Symmetry"("Type of Symmetry"=w2025, "Image Src"=w2026) -> ("Image Dst Out"=→"Detection Laser Y":T2)  [unwired: 3 in, 1 out]
        n680 = call "IMAQ Set Simple Calibration"("Calibration Axis Info"=T31 {"Origin Pixel"={"X"=0.0, "Y"=0.0}, "Angle Relative to Horizontal (deg)"=0.0, "Axis Reference"=0}, "Grid Descriptor"=T32 {"X Step"=0.3, "Y Step"=0.3, "Unit"=enum."Undefined"}, "Image"=w2053) -> ("Calibrated Image"=→"APD 1":T2)  [unwired: 7 in, 1 out]
        n681 = call "IMAQ Set Simple Calibration"("Calibration Axis Info"=T31 {"Origin Pixel"={"X"=0.0, "Y"=0.0}, "Angle Relative to Horizontal (deg)"=0.0, "Axis Reference"=0}, "Grid Descriptor"=T32 {"X Step"=0.3, "Y Step"=0.3, "Unit"=enum."Undefined"}, "Image"=w1994) -> ("Calibrated Image"=→"APD 2":T2)  [unwired: 7 in, 1 out]
      }
    }
    n682 = Subtract(x=w947, y="APD 2 Offset") -> (x-y=w944:waveform(dbl))
    n683 = Subtract(x=w949, y="APD 1 Offset") -> (x-y=w945:waveform(dbl))
    n684 = Index Array(array=w964, index=3) -> (element=w1033:waveform(dbl))
    n685 = Index Array(array=w964, index=6) -> (element=w1030:waveform(dbl))
    n686 = Build Array(w945, w944) -> (→"APD Chart":waveform(dbl)[])
    n687 = Array Size(array=w1022) -> (size(s)=w1077:i32)
    n688 = call <vilib>:"Std Deviation and Variance.vi"("X"=w957) -> ("standard deviation"=w956:dbl)  [unwired: 1 in, 2 out]
    n689 = Add Array Elements(numeric array=w957) -> (sum=w959:u32)
    n690 = Add Array Elements(numeric array=w1022) -> (sum=w1087:u32)
    n691 = call <vilib>:"Std Deviation and Variance.vi"("X"=w1022) -> ("standard deviation"=w1021:dbl)  [unwired: 1 in, 2 out]
    n692 = Divide(x="T1 offset_x (mV)", y=1000.0) -> (x/y=w1034:dbl)
    n693 = Divide(x=w956, y=w955) -> (x/y=w952:dbl)
    "Rate sigma (Hz) 2" <- w952
    n694 = Multiply(x=w955, y=w1077) -> (x*y=w958:dbl)
    "Int. Time (s)" <- w958
    n695 = Divide(x=w959, y=w958) -> (x/y=w953:dbl)
    "APD 2 Rate (Hz)" <- w953
    n696 = Divide(x=w1087, y=w958) -> (x/y=w1019:dbl)
    "APD 1 Rate (Hz)" <- w1019
    n697 = Divide(x=w1021, y=w955) -> (x/y=w1020:dbl)
    "Rate sigma (Hz)" <- w1020
    n698 = Divide(x=w952, y=w953) -> (x/y=→"Sigma/Mean 2":dbl)
    n699 = Divide(x=w1020, y=w1019) -> (x/y=→"Sigma/Mean":dbl)
    n700 = Divide(x="T2 offset_x (mV)", y=1000.0) -> (x/y=w1032:dbl)
    n701 = case shown="0, Default" "Calibration" {
      tunnel: "T1 alpha_x (nm/V)" -> [_ w1952 w1973]
      tunnel: "T1 kappa_x (pN/nm)" -> [_ _ w1963]
      tunnel: "T2 alpha_x (nm/V)" -> [_ w1951 w1971]
      tunnel: "T2 kappa_x (pN/nm)" -> [_ _ w1964]
      tunnel: w1033 -> [w1934 w1949 w1969]
      tunnel: w1030 -> [w1933 w1947 w1967]
      tunnel: [w1934 w1946 w1966] -> w1063
      tunnel: [w1933 w1945 w1965] -> w1062
      tunnel: ["T1 X (V)" ("Label.Text") "T1 X (nm)" ("Label.Text") "T1 X (pN)" ("Label.Text")] -> w1051
      tunnel: ["T2 X (V)" ("Label.Text") "T2 X (nm)" ("Label.Text") "T2 X (pN)" ("Label.Text")] -> w1050
      tunnel: ["Position (V)" ("Label.Text") "Position (nm)" ("Label.Text") "Force (pN)" ("Label.Text")] -> w1052
      tunnel: w1032 -> [_ w1937 w1956]
      tunnel: w1034 -> [_ w1940 w1958]
      tunnel: ["Mean (V)" ("Label.Text") "Mean (nm)" ("Label.Text") "Mean (pN)" ("Label.Text")] -> w1047
      tunnel: ["Difference (V)" ("Label.Text") "Difference (nm)" ("Label.Text") "Difference (pN)" ("Label.Text")] -> w972
      frame 0, Default {
      }
      frame 1 {
        n702 = Unbundle By Name(w1949) -> ("Y"=w1953:dbl[])
        n703 = Unbundle By Name(w1947) -> ("Y"=w1938:dbl[])
        n704 = Subtract(x=w1953, y=w1940) -> (x-y=w1941:dbl[])
        n705 = Subtract(x=w1938, y=w1937) -> (x-y=w1939:dbl[])
        n706 = Multiply(x=w1939, y=w1951) -> (x*y=w1948:dbl[])
        n707 = Multiply(x=w1952, y=w1941) -> (x*y=w1950:dbl[])
        n708 = Bundle By Name(cluster=w1947, "Y"=w1948) -> (w1945:waveform(dbl))
        n709 = Bundle By Name(cluster=w1949, "Y"=w1950) -> (w1946:waveform(dbl))
      }
      frame 2 {
        n710 = Unbundle By Name(w1969) -> ("Y"=w1974:dbl[])
        n711 = Unbundle By Name(w1967) -> ("Y"=w1972:dbl[])
        n712 = Subtract(x=w1972, y=w1956) -> (x-y=w1957:dbl[])
        n713 = Subtract(x=w1974, y=w1958) -> (x-y=w1959:dbl[])
        n714 = Compound Arithmetic op=MULTIPLY(w1957, w1971, w1964) -> (w1968:dbl[])
        n715 = Compound Arithmetic op=MULTIPLY(w1963, w1973, w1959) -> (w1970:dbl[])
        n716 = Bundle By Name(cluster=w1967, "Y"=w1968) -> (w1965:waveform(dbl))
        n717 = Bundle By Name(cluster=w1969, "Y"=w1970) -> (w1966:waveform(dbl))
      }
    }
    n718 = feedback-in #17("Calibration") -> ()
    n719 = feedback #17(u16 1 ("Calibration")) -> (w1054:u16)
    n720 = Not Equal?(x=w1054, y="Calibration") -> (x != y?=w1010:bool)
    n721 = Unbundle By Name(w1033) -> ("Y"=w1036:dbl[])
    n722 = Unbundle By Name(w1030) -> ("Y"=w1039:dbl[])
    n723 = Subtract(x=w1036, y=w1034) -> (x-y=w1037:dbl[])
    n724 = Subtract(x=w1039, y=w1032) -> (x-y=w1038:dbl[])
    n725 = Multiply(x=w1038, y="T2 alpha_x (nm/V)") -> (x*y=w1029:dbl[])
    n726 = Multiply(x="T1 alpha_x (nm/V)", y=w1037) -> (x*y=w1028:dbl[])
    n727 = Multiply(x=w1062, y=-1.0) -> (x*y=w1041:waveform(dbl))
    n728 = case shown="True" "Read Lateness and Rel Phase" {
      tunnel: w863 -> [w1509 w1531]
      tunnel: w862 -> [w1510 w1530]
      tunnel: [w1509 w1529] -> w1025
      tunnel: [w1510 w1528] -> w1024
      frame False {
      }
      frame True {
        n729 = xnode "Read/Write Control"("FPGA VI Reference In"=w1531, "error in"=w1530) -> ("FPGA VI Reference Out"=w1529:T20, "error out"=w1528:errorcluster, "GI Relative phase"=→"GI relative phase":i16, "Relative phase"=→"Relative phase (AI1)":i16, "AI Late Counter"=→"Late Counter (AI1)":u16, "GI Late Counter"=→"GI Late Counter":u16, "MCL Late Counter"=→"MCL Late Counter":u16, "MCL Relative Phase"=→"Relative Phase (MCL)":i16, "APD Acq Relative Phase"=→"APD Acq Relative Phase":i16, "APD 1 Gate Relative Phase"=→"APD 1 Gate Relative Phase":i16, "APD 2 Gate Relative Phase"=→"APD 2 Gate Relative Phase":i16, "APD Acq Late Counter"=→"APD Acq Late Counter":u16, "APD 1 Gate Late Counter"=→"APD 1 Gate Late Counter":u16, "APD 2 Gate Late Counter"=→"APD 2 Gate Late Counter":u16, "Green FB Relative Phase"=→"Relative phase (Green FB)":i16, "GI Relative phase 2"=→"GI relative phase 2":i16, "GI Late Counter 2"=→"GI Late Counter 2":u16, "Trap Pos FIFO Timeout"=→"Trap Pos FIFO Timeout":u16, "Trap AI FIFO Timeout"=→"Trap AI FIFO Timeout":u16)